vi "rydberg_trigger_snap_2014_8_20_joe.vi"() -> ()   [LabVIEW 2013] (continued)
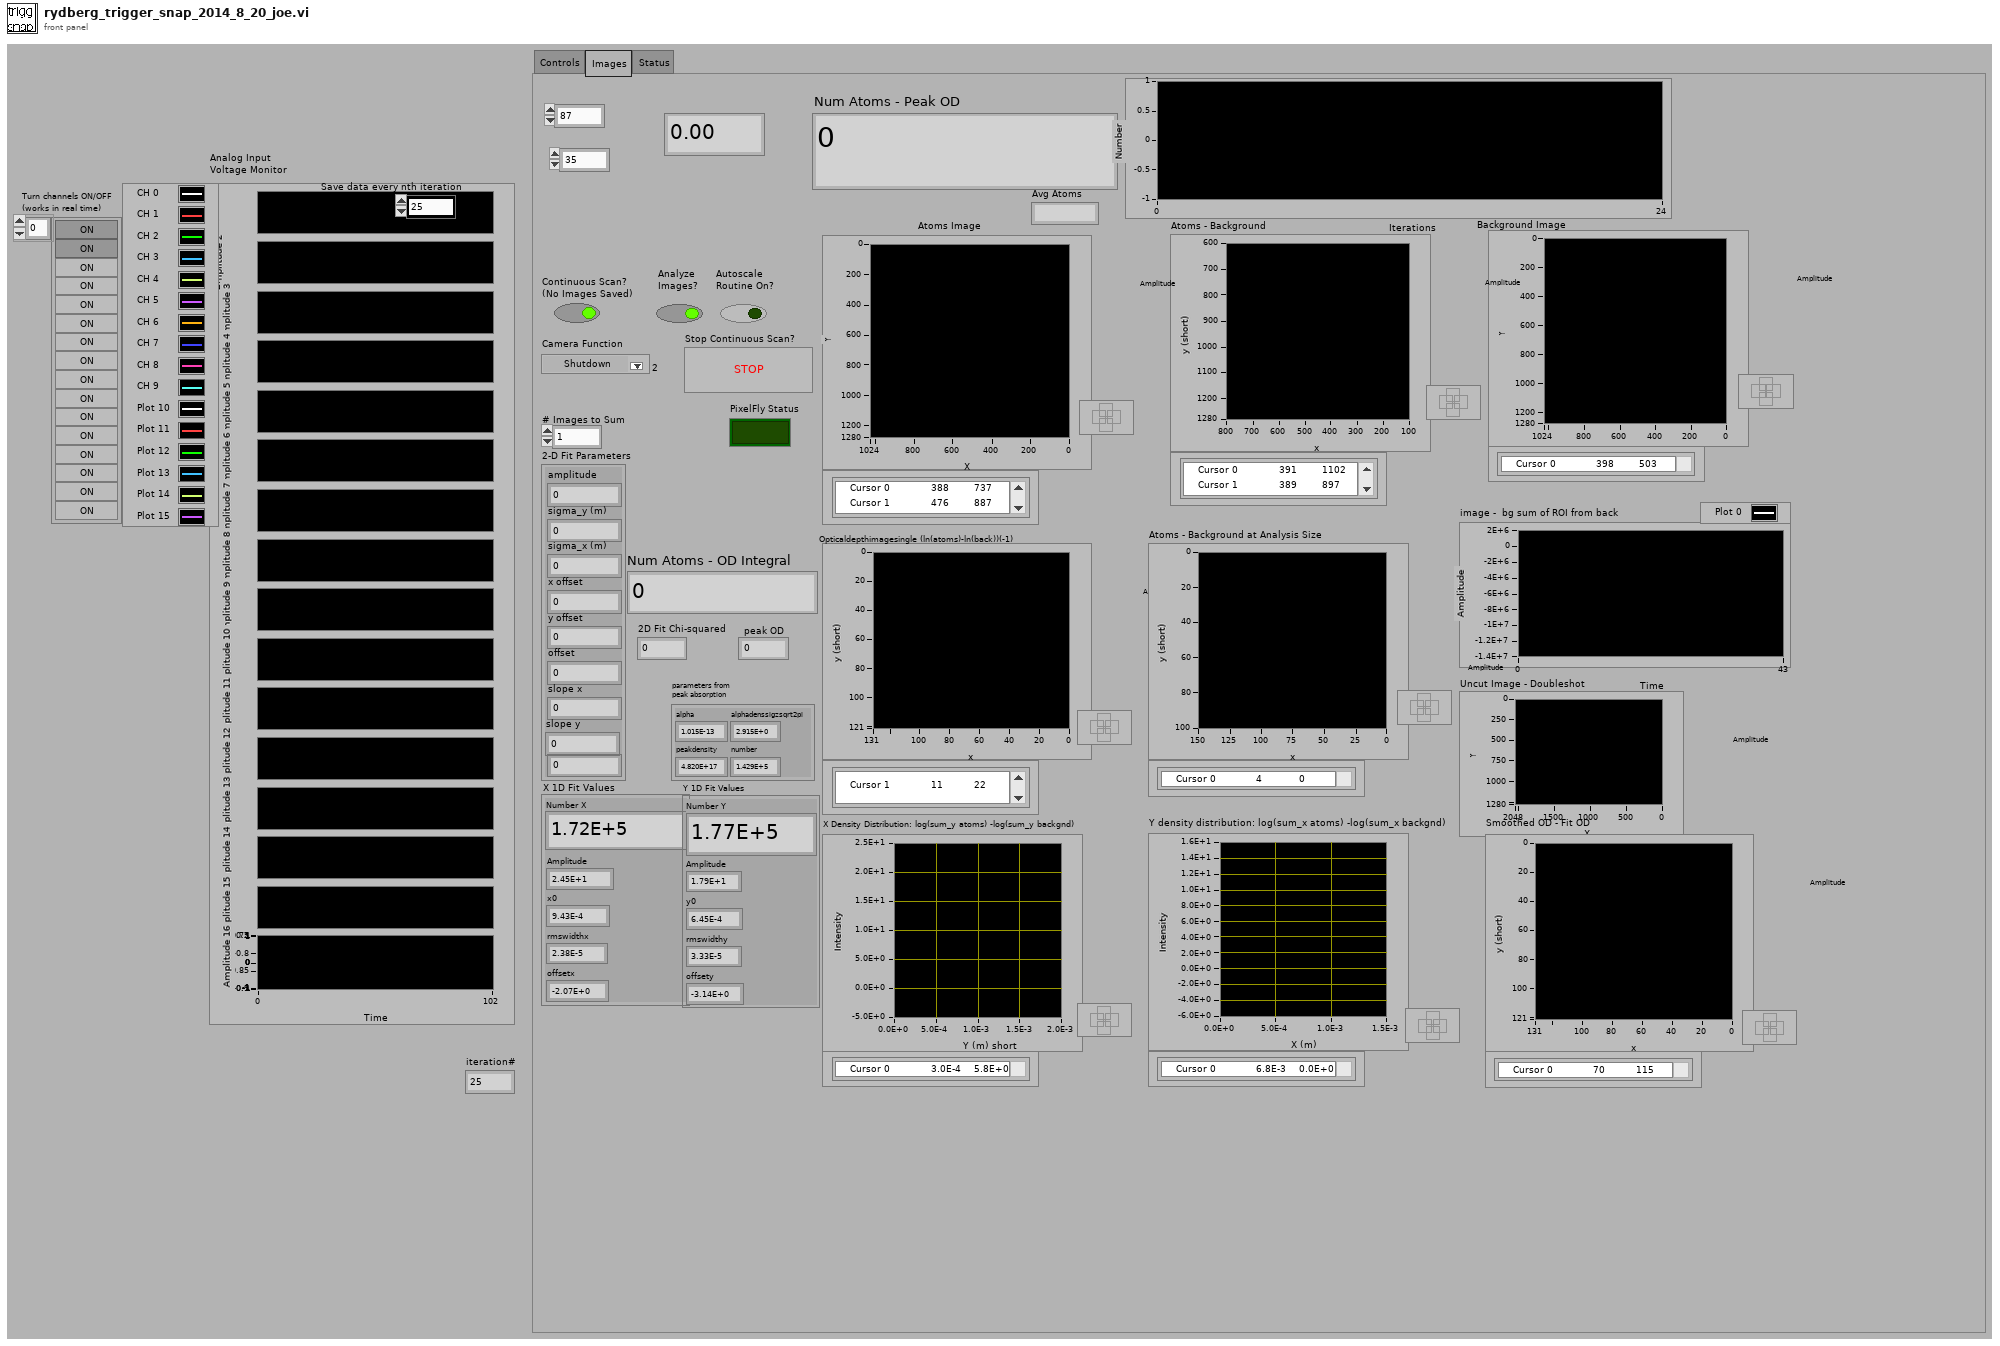
[diagram p1: front panel]
types:
  T1 = cluster{"data[0]":dbl, "data[1]":dbl, "data[2]":dbl, "data[3]":dbl, "data[4]":dbl, "data[5]":dbl, "data[6]":dbl, "data[7]":dbl, "data[8]":dbl, "data[9]":dbl, "data[10]":dbl, "data[11]":dbl, "data[12]":dbl, "data[13]":dbl, "data[14]":dbl, "data[15]":dbl}
  T2 = cluster{"Col Start":i32, "Col Stop":i32, "Row Start":i32, "Row stop":i32}
  T3 = typedef "camera_controls.ctl" = cluster{"Acquisition Mode":T4, "Trigger Mode":T5, "Frame \nTransfer":bool, "Exposure Time (s)":sgl, "Accumulation Cycle Time (s)":sgl, "# Accumulations":i32, "# Kinetics":i32, "Kinetic Cycle Time (s)":sgl}
  T4 = typedef "AcquisitionMode_mode typedef.ctl" = enum16{"Reserved (0)", "Single Scan", "Accumulate", "Kinetics", "Fast Kinetics", "Run Till Abort", "Reserved (6)", "Reserved (7)", "Reserved (8)", "Time Delayed Integration"}
  T5 = typedef "TriggerMode_mode typedef.ctl" = enum16{"Internal", "External", "N/A (2)", "N/A (3)", "N/A (4)", "N/A (5)", "External Start", "External Exposure (Bulb)", "N/A (8)", "External FVB EM", "Software", "N/A (11)", "External Charge Shifting"}
  T6 = cluster{"alpha":dbl, "peakdensity":dbl, "alphadenssigzsqrt2pi":sgl, "number":dbl}
  T7 = cluster{"Amplitude":dbl, "y0":dbl, "rmswidthy":dbl, "offsety":dbl, "Number Y":dbl}
  T8 = cluster{"Amplitude":dbl, "x0":dbl, "rmswidthx":dbl, "offsetx":dbl, "Number X":dbl}
  T9 = cluster{"amplitude":dbl, "sigma_y (m)":dbl, "sigma_x (m)":dbl, "x offset":dbl, "y offset":dbl, "offset":dbl, "slope x":dbl, "slope y":dbl, dbl}
  T10 = cluster{"Write":bool, "Write done":bool, "Queued":bool, "Cancelled":bool, "Select":bool, "Select done":bool, "Burst":bool, "Size":bool, "Event":bool, "Timeout":bool, "Open":i32, "Map":i32, "Exposure":i32[], "Offset":i32[], "Size":i32[], "Transfer":i32[], "Total Size":i32}
  T11 = cluster{"xpixels":i32, "ypixels":i32, "# VS Speeds":i32, "VS Speed (us)":sgl, "Temperature Stable":bool, "Temperature (C)":i32}
  T12 = cluster{"amplitudey":dbl, "temperaturey":dbl, "alphay":dbl, "offsety":dbl, "numbery":dbl, "peakdensityy":dbl, "centery":dbl}
  T13 = cluster{"amplitudex":dbl, "temperaturex":dbl, "alphax":dbl, "offsetx":dbl, "numberx":dbl, "peakdensityx":dbl, "centerx":dbl}
  T14 = cluster{"Initalize Error Code":u32, "GetDetector Error Code":u32, "Get#VSSpeeds Error Code":u32, "Set VS Speed Error":u32, "CoolerOn Error Code":u32, "GetTemperature Error Code":u32, "Shutdown Error Code":u32}
  T15 = cluster{"ccdxsize":i32, "ccdy":i32, "pictx":i32, "picty":i32, "bitspixel":i32}
  T16 = cluster{"Sample Interleave":dbl, "Pixel Size (m)":dbl, i32, "Cut Borders":dbl, "Number for Scale":dbl, "Limit":dbl, "Number of Pixels to Smooth":dbl}
  T17 = cluster{"abscrosssection":dbl, "peakdensity":dbl, "twosizeoneoverezabsxsecdens":dbl, "number":dbl}
  T18 = cluster{"Amplitude":dbl, "x0":dbl, "rmswidthx":dbl, "offsetx":dbl, "numberx":dbl}
  T19 = cluster{"Amplitude":dbl, "y0":dbl, "rmswidthy":dbl, "offsety":dbl, "numbery":dbl}
  T20 = cluster{"amplitude":dbl, "sigma_y (m)":dbl, "sigma_x (m)":dbl, "row offset (pixel #)":dbl, "col offset (pixel #)":dbl, "offset":dbl, "slope x":dbl, "slope y":dbl, dbl}
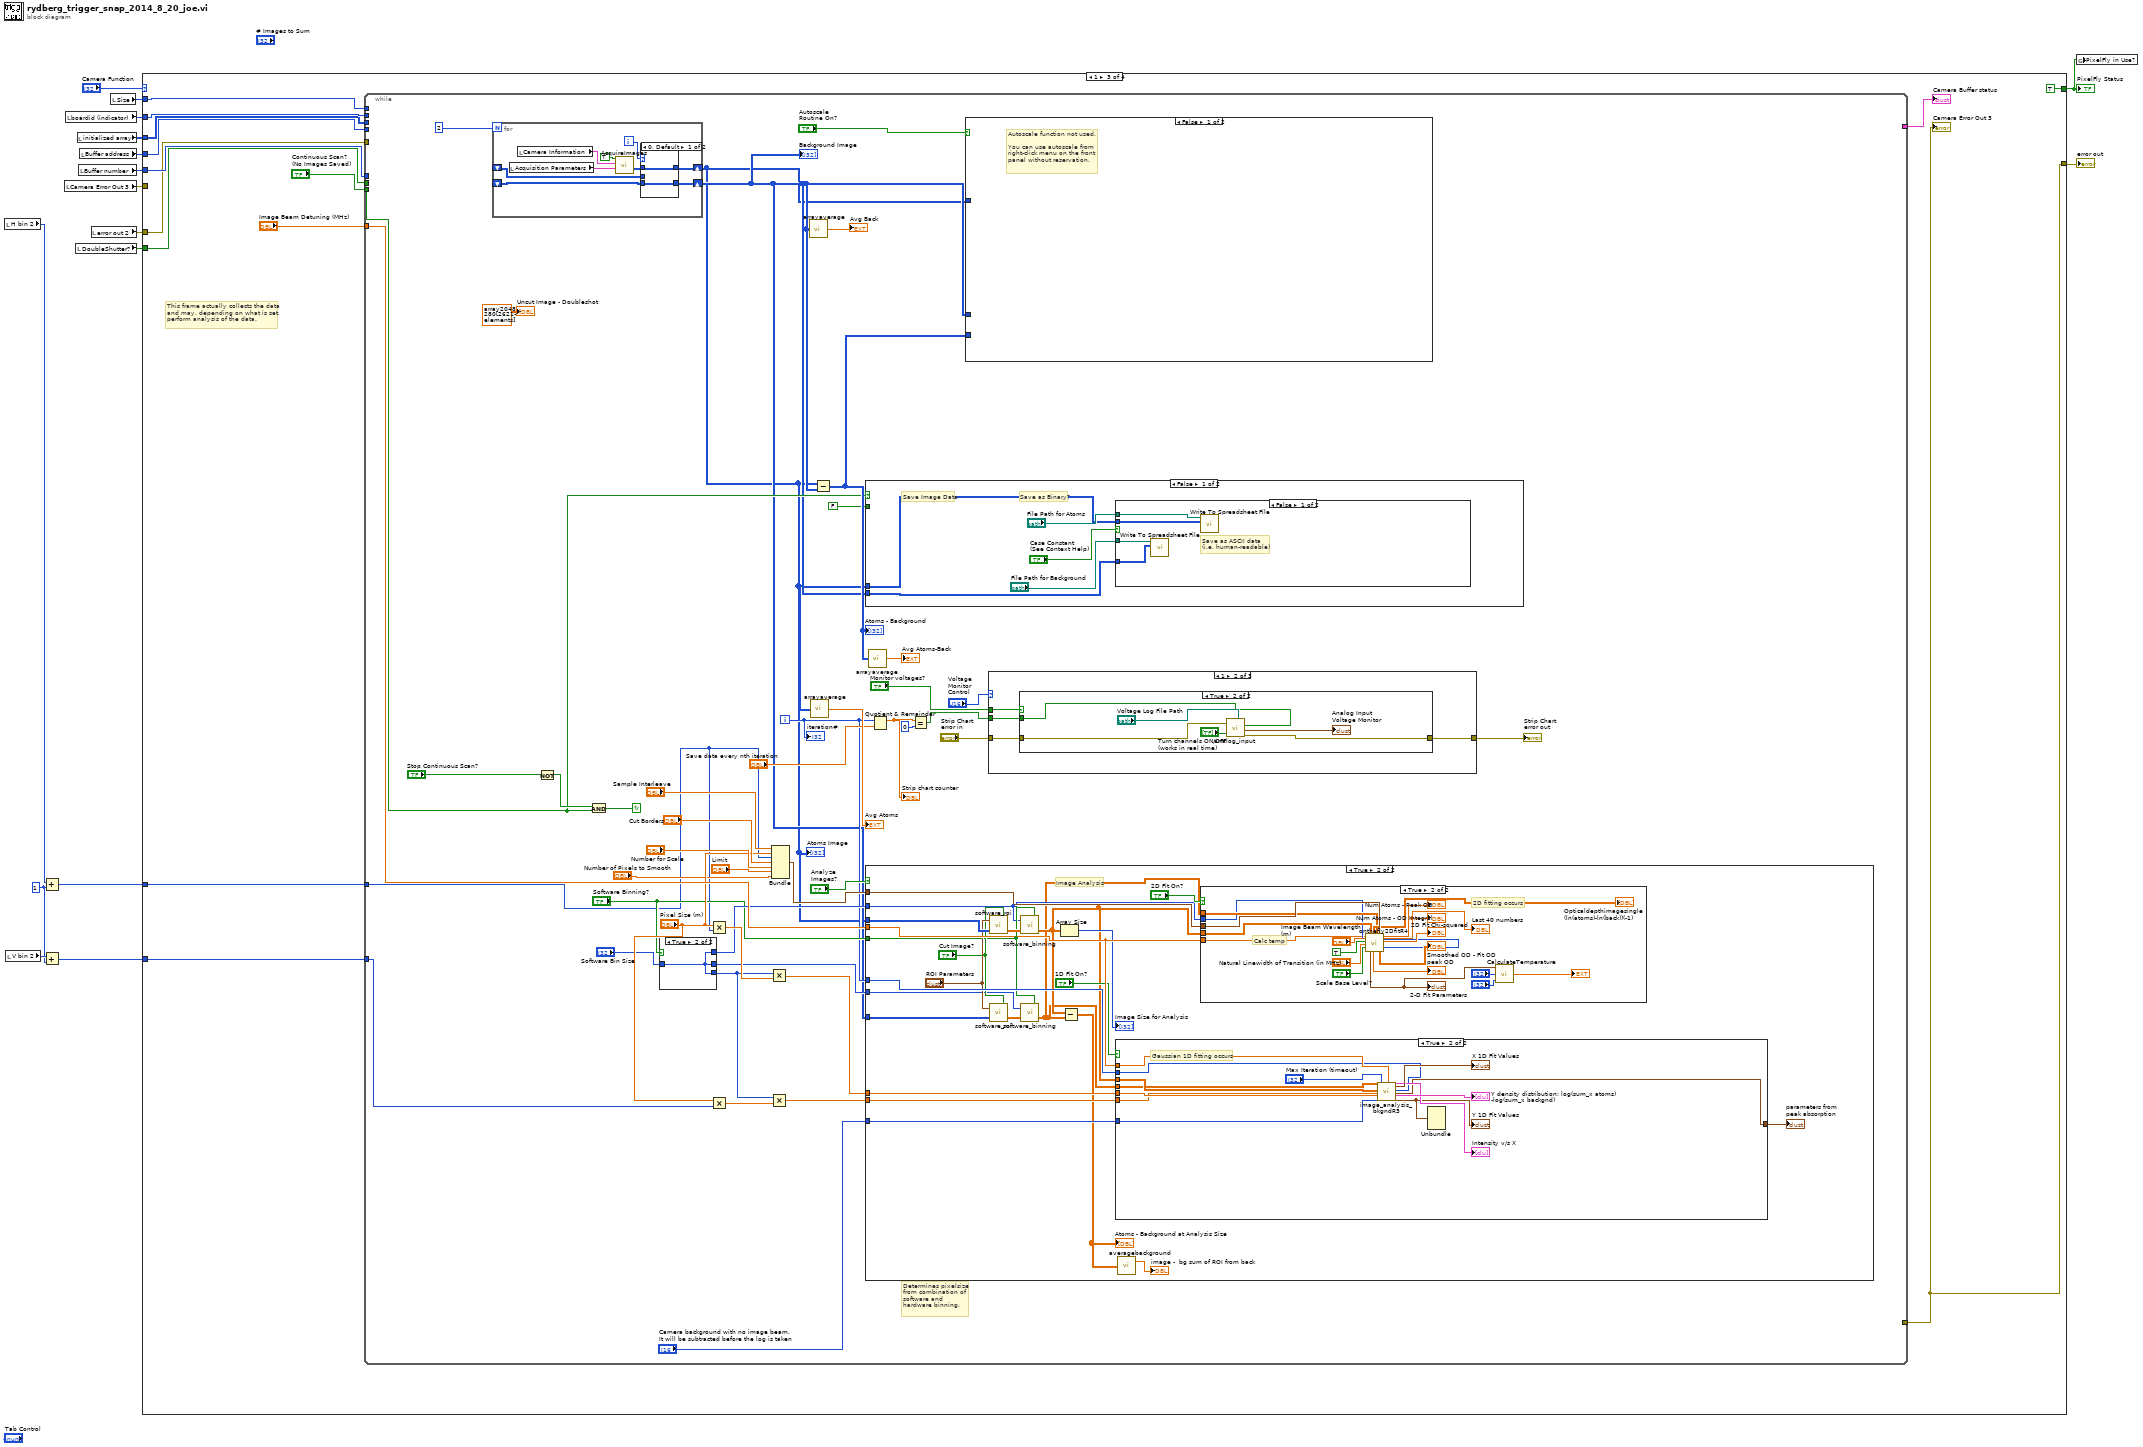
[diagram p0: block diagram]
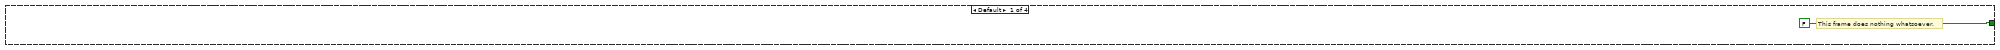
[diagram p2: hidden frame]
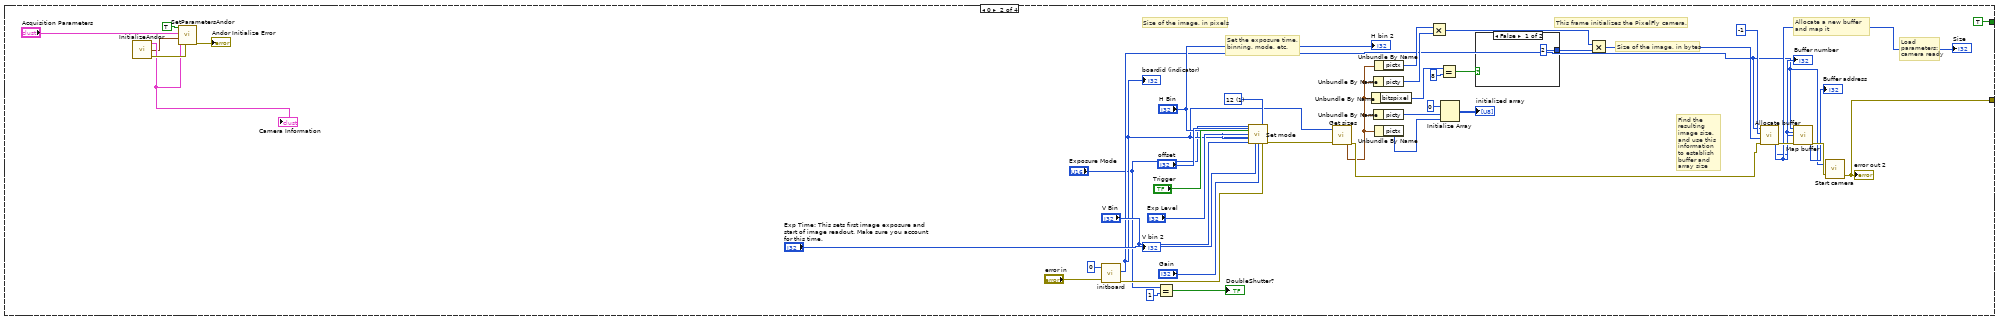
[diagram p3: hidden frame]
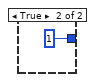
[diagram p4: hidden frame]
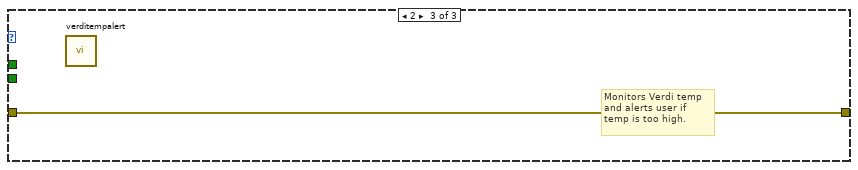
[diagram p8: hidden frame]
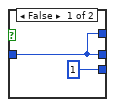
[diagram p9: hidden frame]
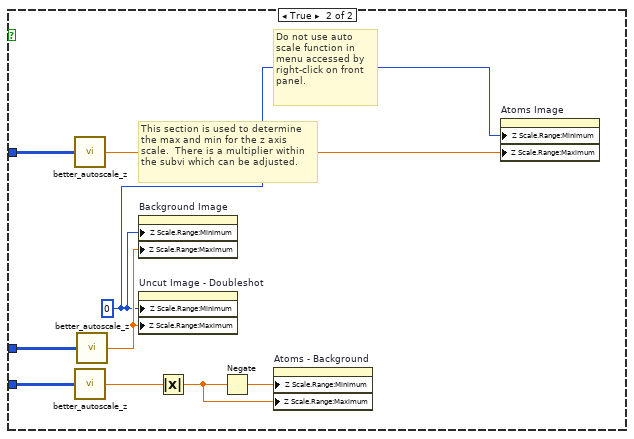
[diagram p10: hidden frame]
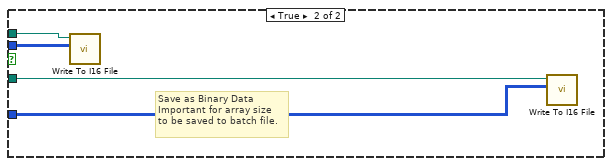
[diagram p11: hidden frame]
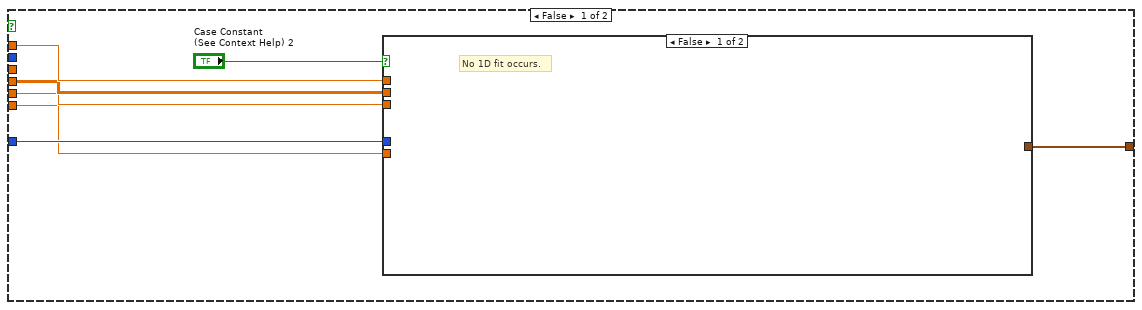
[diagram p15: hidden frame]
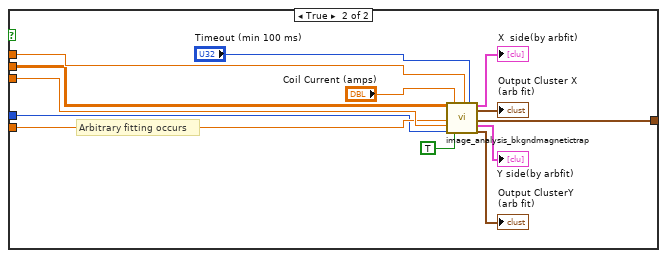
[diagram p16: hidden frame]
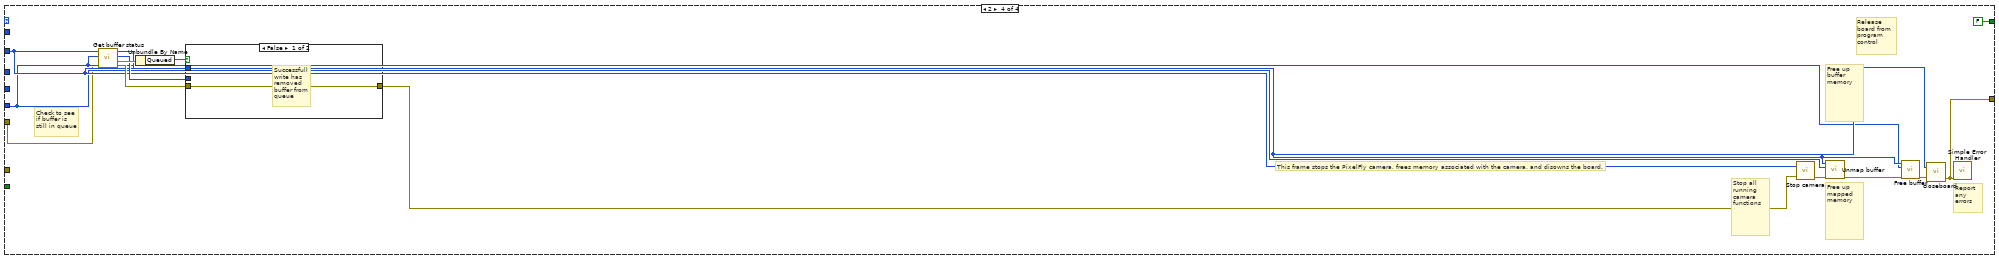
[diagram p17: hidden frame]
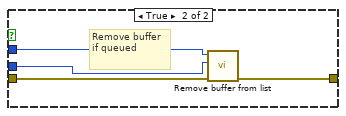
[diagram p18: hidden frame]
diagram:
  w5 = 1
  n1 = local read "H bin 2"() -> (w8:i32)
  n2 = local read "V bin 2"() -> (w6:i32)
  n3 = Add(x=w8, y=w5) -> (x+y=w7:i32)
  n4 = Add(x=w6, y=w5) -> (x+y=w4:i32)
  n5 = local read "Camera Error Out 3"() -> (w14:errorcluster)
  n6 = local read "boardid (indicator)"() -> (w9:i32)
  n7 = local read "DoubleShutter?"() -> (w2:bool)
  n8 = local read "initialized array"() -> (w3:u8[][])
  n9 = local read "Buffer number"() -> (w11:i32)
  n10 = local read "Buffer address"() -> (w13:i32)
  n11 = local read "error out 2"() -> (w15:errorcluster)
  n12 = local read "Size"() -> (w12:i32)
  n13 = case shown="1" "Camera Function" {
    tunnel: w15 -> [_ _ w64 _]
    tunnel: w14 -> [_ _ _ w249]
    tunnel: w13 -> [_ _ w75 _]
    tunnel: w12 -> [_ _ w74 _]
    tunnel: w11 -> [_ _ w72 w250]
    tunnel: w7 -> [_ _ w70 _]
    tunnel: w4 -> [_ _ w71 _]
    tunnel: [_ w32 w69 w252] -> w10
    tunnel: w9 -> [_ _ w68 w251]
    tunnel: w3 -> [_ _ w67 _]
    tunnel: w2 -> [_ _ w66 _]
    tunnel: [FALSE TRUE TRUE FALSE] -> w1
    frame Default {
      # "This frame does nothing whatsoever."
    }
    frame 0 {
      w43 = 1 items=["8", "12"] ("bits/pixel")
      # "This frame initializes the PixelFly camera."
      # "Load parameters: camera ready"
      # "Allocate a new buffer and map it"
      # "Set the exposure time, binning, mode, etc."
      # "Find the resulting image size, and use this information to establish buffer and array size"
      # "Size of the image, in pixels"
      # "Size of the image, in bytes"
      n14 = call "InitializeAndor.vi"() -> ("error out"=w23:errorcluster, "Andor Initialization Error Codes"=w21:T14, "Camera Information"=w22:T11)  [unwired: 3 in]
      "Camera Information" <- w22
      n15 = call "SetParametersAndor.vi"("Error In"=w23, "Camera Information"=w22, "Andor Initialization Error Codes"=w21, "Acquisition Parameters"="Acquisition Parameters", "Pre Initialized?"=TRUE) -> ("error out"=→"Andor Initialize Error":errorcluster)  [unwired: 4 in, 2 out]
      n16 = call "initboard.vi"("boardid in"=0, "error in (no error)"="error in") -> ("boardid"=w29:i32, "error out"=w28:errorcluster)  [unwired: 2 in, 1 out]
      "boardid (indicator)" <- w29
      n17 = Equal?(x="Exposure Mode", y=1) -> (x = y?=→"DoubleShutter?":bool)
      n18 = call "Set mode.vi"("Exposure mode"="Exposure Mode", "Handle in"=w29, "offset"="offset", "bits/pixel"=w43, "trigger"="Trigger", "exp level"="Exp Level", "H bin"="H Bin", "V bin"="V Bin", "exp time"="Exp Time: This sets first image exposure and start of image readout. Make sure you account for this time.", "gain"="Gain", "error in (no error)"=w28) -> ("error out"=w56:errorcluster)  [unwired: 4 in]
      n19 = call "Get sizes.vi"("Handle in"=w29, "error in (no error)"=w56) -> ("Picture parameters"=w42:T15, "error out"=w47:errorcluster)  [unwired: 1 in, 2 out]
      n20 = Unbundle By Name(w42) -> ("bitspixel"=w53:i32)
      n21 = Unbundle By Name(w42) -> ("picty"=w54:i32)
      n22 = Unbundle By Name(w42) -> ("picty"=w35:i32)
      n23 = Unbundle By Name(w42) -> ("pictx"=w55:i32)
      n24 = Unbundle By Name(w42) -> ("pictx"=w34:i32)
      n25 = Multiply(x=w55, y=w54) -> (x*y=w50:i32)
      n26 = Equal?(x=w53, y=8) -> (x = y?=w51:bool)
      n27 = Initialize Array(u8 0 ("16 bit integers"), w35, w34) -> (→"initialized array":u8[][])
      n28 = case shown="False" w51 {
        tunnel: [2 1] -> w49
        frame False {
        }
        frame True {
        }
      }
      n29 = Multiply(x=w50, y=w49) -> (x*y=w48:i32)
      n30 = call "Allocate buffer.vi"("error in (no error)"=w47, "Size request"=w48, "Buffer request"=-1, "Handle in"=w29) -> ("error out"=w45:errorcluster, "Size"=w40:i32, "Buffer number"=w39:i32)  [unwired: 1 out]
      "Size" <- w40
      "Buffer number" <- w39
      n31 = call "Map buffer.vi"("Handle in"=w29, "Buffer in"=w39, "size"=w40, "error in (no error)"=w45) -> ("Buffer address"=→"Buffer address":i32, "error out"=w41:errorcluster)  [unwired: 8 in, 2 out]
      n32 = call "Start camera.vi"("Handle in"=w29, "error in (no error)"=w41) -> ("error out"=w32:errorcluster)  [unwired: 2 out]
      "error out 2" <- w32
      "H bin 2" <- "H Bin"
      "V bin 2" <- "V Bin"
    }
    frame 1 {
      # "This frame actually collects the data\nand may, depending on what is set,\nperform analysis of the data."
      n33 = while {
        tunnel: "Image Beam Detuning (MHz)" -> [w121]
        tunnel: w64 -> [_]
        tunnel: "Continuous Scan?\n(No Images Saved)" -> [w82]
        tunnel: [_] -> w69
        tunnel: w75 -> [_]
        tunnel: w68 -> [_]
        tunnel: w74 -> [_]
        tunnel: w72 -> [_]
        tunnel: [_] -> w73
        tunnel: w71 -> [w117]
        tunnel: w70 -> [w86]
        tunnel: w67 -> [_]
        tunnel: w66 -> [_]
        i -> [w87]
        stop <- w120 continue-if-true
        # "Determines pixelsize\nfrom combination of\nsoftware and\nhardware binning."
        n34 = for {
          N: 2 -> [_]
          shift-right: [w126] -> w78
          shift-left: _ -> [w123]
          shift-right: [w124] -> w80
          shift-left: _ -> [w122]
          i -> [w127]
          n35 = local read "Acquisition Parameters"() -> (w129:T3)
          n36 = local read "Camera Information"() -> (w128:T11)
          n37 = call "AcquireImages.vi"("Acquisition Parameters"=w129, "Camera Information 2"=w128, "Pre Initialized?"=TRUE) -> ("Intensity Graph"=w125:i32[][])  [unwired: 7 in, 1 out]
          n38 = case shown="0, Default" w127 {
            tunnel: [w132 w133] -> w126
            tunnel: w125 -> [w132 w134]
            tunnel: [w131 w134] -> w124
            tunnel: w123 -> [_ w133]
            tunnel: w122 -> [w131 _]
            frame 0, Default {
            }
            frame 1 {
            }
          }
        }
        "Atoms Image" <- w78
        "Background Image" <- w80
        n39 = Not(x="Stop Continuous Scan?") -> (.not. x?=w118:bool)
        n40 = And(x=w118, y=w82) -> (x .and. y?=w120:bool)
        n41 = case shown="True" "Software Binning?" {
          tunnel: [w149 w150] -> w98
          tunnel: "Software Bin Size" -> [w149 w150]
          tunnel: [w149 w150] -> w96
          tunnel: [1 w150] -> w95
          frame False {
          }
          frame True {
          }
        }
        n42 = Multiply(x="Pixel Size (m)", y=w86) -> (x*y=w111:dbl)
        n43 = Multiply(x="Pixel Size (m)", y=w117) -> (x*y=w110:dbl)
        n44 = Multiply(x=w95, y=w111) -> (x*y=w107:dbl)
        n45 = Multiply(x=w95, y=w110) -> (x*y=w109:dbl)
        n46 = Bundle("Sample Interleave"="Sample Interleave", "Pixel Size (m)"="Pixel Size (m)", w86, "Cut Borders"="Cut Borders", "Number for Scale"="Number for Scale", "Limit"="Limit", "Number of Pixels to Smooth"="Number of Pixels to Smooth") -> (w108:T16)  [unwired: 1 in]
        n47 = call "arrayaverage.vi"("Array int 32"=w80) -> ("Average"=→"Avg Back":ext)
        n48 = call "arrayaverage.vi"("Array int 32"=w78) -> ("Average"=→"Avg Atoms":ext)
        n49 = Subtract(x=w78, y=w80) -> (x-y=w106:i32[][])
        "Atoms - Background" <- w106
        n50 = case shown="False" w82 {
          tunnel: w78 -> [w161 _]
          tunnel: w80 -> [w160 _]
          tunnel: FALSE -> [_ _]
          frame False {
            # "Save as Binary?"
            # "Save Image Data"
            n51 = case shown="False" "Case Constant\n(See Context Help)" {
              tunnel: "File Path for Atoms" -> [w168 w172]
              tunnel: "File Path for Background" -> [w167 w171]
              tunnel: w161 -> [w166 w169]
              tunnel: w160 -> [w165 w170]
              frame False {
                # "Save as ASCII data\n(i.e. human-readable)"
                n52 = call-poly <vilib>:"Write To Spreadsheet File.vi"("2D data"=w165, "file path (dialog if empty)"=w167) -> ()  [unwired: 6 in, 1 out]
                n53 = call-poly <vilib>:"Write To Spreadsheet File.vi"("2D data"=w166, "file path (dialog if empty)"=w168) -> ()  [unwired: 6 in, 1 out]
              }
              frame True {
                # "Save as Binary Data\nImportant for array size\nto be saved to batch file."
                n54 = call <vilib>:"Write To I16 File.vi"("2D array"=w169, "file path (dialog if empty)"=w172) -> ()  [unwired: 5 in, 1 out]
                n55 = call <vilib>:"Write To I16 File.vi"("2D array"=w170, "file path (dialog if empty)"=w171) -> ()  [unwired: 5 in, 1 out]
              }
            }
          }
          frame True {
            # "Don't Save Data\nWhen Continous"
          }
        }
        n56 = case shown="True" "Analyze \nImages?" {
          tunnel: w107 -> [_ w185]
          tunnel: w109 -> [_ w184]
          tunnel: "Camera background with no image beam.\nIt will be subtracted before the log is taken" -> [_ w195]
          tunnel: w121 -> [_ w193]
          tunnel: w87 -> [_ w194]
          tunnel: w108 -> [_ w192]
          tunnel: w78 -> [_ w189]
          tunnel: w80 -> [_ w186]
          tunnel: w96 -> [_ w177]
          tunnel: "Software Binning?" -> [_ w180]
          tunnel: w98 -> [_ w179]
          frame False {
            # "Perform No Analysis"
            # "No analysis done."
          }
          frame True {
            # "Image Analysis"
            n57 = call "software_roi.vi"("Cut image?"="Cut Image?", "Input Array"=w189, "ROI Controls"="ROI Parameters") -> ("output array"=w182:sgl[][])
            n58 = call "software_roi.vi"("Cut image?"="Cut Image?", "Input Array"=w186, "ROI Controls"="ROI Parameters") -> ("output array"=w181:sgl[][])
            n59 = call "software_binning.vi"("Bin image?"=w180, "Input Array"=w182, "bin size"=w177) -> ("Binned Array"=w178:dbl[][])
            n60 = call "software_binning.vi"("Bin image?"=w180, "Input Array"=w181, "bin size"=w179) -> ("Binned Array"=w176:dbl[][])
            n61 = Array Size(array=w178) -> (size(s)=→"Image Size for Analysis":i32[])
            n62 = Subtract(x=w178, y=w176) -> (x-y=w175:dbl[][])
            "Atoms - Background at Analysis Size" <- w175
            n63 = case shown="True" "1D Fit On?" {
              tunnel: w176 -> [w219 w237]
              tunnel: w195 -> [w221 w242]
              tunnel: w193 -> [w220 w246]
              tunnel: w178 -> [_ w238]
              tunnel: w194 -> [_ w241]
              tunnel: w185 -> [w217 w240]
              tunnel: w184 -> [w216 w239]
              tunnel: [w215 w235] -> w173
              frame False {
                n64 = case shown="False" "Case Constant\n(See Context Help) 2" {
                  tunnel: w217 -> [_ w233]
                  tunnel: w216 -> [_ w232]
                  tunnel: w221 -> [_ w231]
                  tunnel: w220 -> [_ w229]
                  tunnel: w219 -> [_ w224]
                  tunnel: [_ w222] -> w215
                  frame False {
                    # "No 1D fit occurs."
                  }
                  frame True {
                    # "Arbitrary fitting occurs"
                    n65 = call "image_analysis_bkgndmagnetictrap.vi"("2D Array In"=w224, "Delta_x (m)"=w232, "Delta_y (m)"=w233, "camera background with no image beam\nIt will be subtracted before the log is taken"=w231, "coilcurrent"="Coil Current (amps)", "take new\nnew image"=TRUE ("take new\nnew image"), "Image beam \nDetuning (MHz)"=w229, "timeout(min 100ms)"="Timeout (min 100 ms)") -> ("X  side"=→"X  side(by arbfit)":cluster{cluster{dbl, dbl}[]}[], "Output Cluster X"=→"Output Cluster X\n(arb fit)":T13, "parameters from\n peak absorption"=w222:T17, "Y side"=→"Y side(by arbfit)":cluster{cluster{dbl, dbl}[]}[], "Output ClusterY"=→"Output ClusterY\n(arb fit)":T12)  [unwired: 5 in, 2 out]
                  }
                }
              }
              frame True {
                # "Gaussian 1D fitting occurs"
                n66 = call "image_analysis_bkgndR3.vi"("Atoms array in"=w238, "BG array in"=w237, "Delta_x (m)"=w239, "Delta_y (m)"=w240, "camera background with no image beam\nIt will be subtracted before the log is taken"=w242, "max iteration"="Max Iteration (timeout)", "Image beam \nDetuning (MHz)"=w246, "Iteration #"=w241) -> ("Intensity v/s X 2"=→"Intensity v/s X":cluster{dbl[], dbl[]}[], "x fit values"=→"X 1D Fit Values":T18, "parameters from \npeak absorption"=w235:T6, "Intensity v/s X"=→"Y density distribution: log(sum_x atoms) -log(sum_x backgnd)":cluster{dbl[], dbl[]}[], "y fit values"=w236:T19)  [unwired: 13 in, 2 out]
                "Y 1D Fit Values" <- w236
                n67 = Unbundle(w236) -> ()  [unwired: 5 out]
              }
            }
            "parameters from \npeak absorption" <- w173
            n68 = call "averagebackground.vi"("Input Array"=w175) -> ("sum of Gaussian"=→"image -  bg sum of ROI from back":dbl)  [unwired: 1 out]
            n69 = case shown="True" "2D Fit On?" {
              tunnel: w178 -> [_ w204]
              tunnel: w193 -> [_ w200]
              tunnel: w192 -> [_ w209]
              tunnel: w176 -> [_ w203]
              tunnel: w177 -> [_ w202]
              frame False {
                # "No 2D fitting occurs"
              }
              frame True {
                # "Calc temp"
                # "2D fitting occurs"
                n70 = call "onthefly2DfitR4.vi"("Detuning in MHz"=w200, "Wavelength (m)"="Image Beam Wavelength (m)", "pass image method"=TRUE, "Natural Linewidth of Transition\n(ion fwhm in MHz)"="Natural Linewidth of Transition (in MHz)", "Scale Base Level?"="Scale Base Level?", "Atoms"=w204, "Background"=w203, "Specifics of Fitting Routines"=w209, "Software bin size"=w202) -> ("2-D Gaussian Fit Parameters"=w196:T20, "opticaldepthimagesingle\n(ln(atoms)-ln(back))(-1)"=→"Opticaldepthimagesingle (ln(atoms)-ln(back))(-1)":dbl[][], "peak OD"=→"peak OD":dbl, "smoothed OD-fit OD"=→"Smoothed OD - Fit OD":dbl[][], "# atoms from peakOD"=→"Num Atoms - Peak OD":dbl, "# atoms from \nODintegral"=→"Num Atoms - OD Integral" →"Last 40 numbers":dbl, "Chi-squared"=→"2D Fit Chi-squared":dbl)  [unwired: 2 in, 2 out]
                "2-D Fit Parameters" <- w196
                n71 = call "CalculateTemperature.vi"("Droptime (ms)"="?", "Isotope"="?", "2-D Fit Parameters"=w196) -> ("Avg. Temp"=→"?":ext)
              }
            }
          }
        }
        n72 = call "arrayaverage.vi"("Array int 32"=w106) -> ("Average"=→"Avg Atoms-Back":ext)
        n73 = Quotient & Remainder(x=w87, y="Save data every nth iteration") -> (x-y*floor(x/y)=w88:dbl)  [unwired: 1 out]
        "Strip chart counter" <- w88
        n74 = Equal?(x=w88, y=0) -> (x = y?=w85:bool)
        n75 = case shown="False" "Autoscale\nRoutine On?" {
          tunnel: w78 -> [_ w159]
          tunnel: w80 -> [_ w157]
          tunnel: w106 -> [_ w155]
          frame False {
            # "Autoscale function not used.\n\nYou can use autoscale from\nright-click menu on the front\npanel without reservation."
          }
          frame True {
            w154 = 0
            # "Do not use auto\nscale function in\nmenu accessed by\nright-click on front\npanel."
            # "This section is used to determine\nthe max and min for the z axis\nscale.  There is a multiplier within\nthe subvi which can be adjusted."
            n76 = call "better_autoscale_z.vi"("Input Array"=w159) -> ("autoscale max"=w158:dbl)
            n77 = call "better_autoscale_z.vi"("Input Array"=w155) -> ("autoscale max"=w153:dbl)
            n78 = call "better_autoscale_z.vi"("Input Array"=w157) -> ("autoscale max"=w156:dbl)
            n79 = property on="Background Image" class="IntGraph (strict)"("Z Scale.Range:Minimum"=w154, "Z Scale.Range:Maximum"=w156) -> ()  [unwired: 2 in, 2 out]
            n80 = property on="Uncut Image - Doubleshot" class="IntGraph (strict)"("Z Scale.Range:Minimum"=w154, "Z Scale.Range:Maximum"=w156) -> ()  [unwired: 2 in, 2 out]
            n81 = Absolute Value(x=w153) -> (abs(x)=w151:dbl)
            n82 = Negate(x=w151) -> (-x=w152:dbl)
            n83 = property on="Atoms - Background" class="IntGraph (strict)"("Z Scale.Range:Minimum"=w152, "Z Scale.Range:Maximum"=w151) -> ()  [unwired: 2 in, 2 out]
            n84 = property on="Atoms Image" class="IntGraph (strict)"("Z Scale.Range:Minimum"=w154, "Z Scale.Range:Maximum"=w158) -> ()  [unwired: 2 in, 2 out]
          }
        }
        n85 = case shown="1" "Voltage\nMonitor\nControl" {
          tunnel: "Strip Chart\nerror in" -> [w135 w139 w147]
          tunnel: [w135 w138 w147] -> w91
          tunnel: "Monitor voltages?" -> [_ w137 _]
          tunnel: w85 -> [_ w136 _]
          frame 0, Default {
          }
          frame 1 {
            n86 = case shown="True" w137 {
              tunnel: w139 -> [w140 w145]
              tunnel: [w140 w144] -> w138
              tunnel: w136 -> [_ w141]
              frame False {
              }
              frame True {
                n87 = call "analog_input.vi"("save values?"=w141, "Voltage Log File Path"="Voltage Log File Path", 5:"Turn channels ON/OFF\n(works in real time)", "error in"=w145) -> ("error out"=w144:errorcluster, "Data display"=→"Analog Input \nVoltage Monitor":T1)  [unwired: 1 out]
              }
            }
          }
          frame 2 {
            # "Monitors Verdi temp\nand alerts user if\ntemp is too high."
            n88 = call "verditempalert.vi"() -> ()  [unwired: 1 in]
          }
        }
        "Strip Chart\nerror out" <- w91
        "Uncut Image - Doubleshot" <- dbl[][] array2048x1280[2621440 elements] ("Uncut Image - Doubleshot")
        "iteration#" <- w87
      }
      "Camera Error Out 3" <- w69
      "Camera Buffer status" <- w73
    }
    frame 2 {
      # "This frame stops the PixelFly camera, frees memory associated with the camera, and disowns the board."
      # "Check to see if buffer is still in queue"
      # "Report any errors"
      # "Release board from program control"
      # "Free up buffer memory"
      # "Free up mapped memory"
      # "Stop all running camera functions"
      n89 = call "Get buffer status.vi"("error in (no error)"=w249, "Buffer request"=w250, "Handle in"=w251) -> ("error out"=w257:errorcluster, "Buffer status"=w258:T10, "Buffer number"=w254:i32, "Handle out"=w253:i32)  [unwired: 1 in]
      n90 = Unbundle By Name(w258) -> ("Queued"=w256:bool)
      n91 = case shown="False" w256 {
        tunnel: w257 -> [w262 w266]
        tunnel: [w262 w265] -> w255
        tunnel: w254 -> [_ w264]
        tunnel: w253 -> [_ w263]
        frame False {
          # "Successfull write has removed buffer from queue"
        }
        frame True {
          # "Remove buffer if queued"
          n92 = call "Remove buffer from list.vi"("error in (no error)"=w266, "Buffer in"=w264, "Handle in"=w263) -> ("error out"=w265:errorcluster)  [unwired: 2 in, 2 out]
        }
      }
      n93 = call "Stop camera.vi"("Handle in"=w251, "error in (no error)"=w255) -> ("error out"=w260:errorcluster)  [unwired: 2 out]
      n94 = call "Unmap buffer.vi"("error in (no error)"=w260, "Buffer in"=w250, "Handle in"=w251) -> ("error out"=w261:errorcluster)  [unwired: 2 in, 2 out]
      n95 = call "Free buffer.vi"("error in (no error)"=w261, "Buffer in"=w250, "Handle in"=w251) -> ("error out"=w259:errorcluster)  [unwired: 2 in, 2 out]
      n96 = call "closeboard.vi"("Handle in"=w251, "error in (no error)"=w259) -> ("error out"=w252:errorcluster)  [unwired: 2 out]
      n97 = call <vilib>:"Simple Error Handler.vi"("error in (no error)"=w252) -> ()  [unwired: 4 in, 5 out]
    }
  }
  "error out" <- w10
  "PixelFly Status" <- w1
  n98 = global write "check_pixelfly_status.vi" "PixelFly in Use?"(w1) -> ()
